vi "FlexMag - 23-03-2023.vi"() -> ()   [LabVIEW 2018] (continued)
        n2608 = Mantissa & Exponent(0:w3782) -> (2:w3784:dbl)  [unwired: 1 out]
        n2609 = Mantissa & Exponent(0:w3768) -> (2:w3770:dbl)  [unwired: 1 out]
        n2610 = Mantissa & Exponent(0:w3822) -> (2:w3824:dbl)  [unwired: 1 out]
        n2611 = Mantissa & Exponent(0:w3819) -> (2:w3817:dbl)  [unwired: 1 out]
        n2612 = Mantissa & Exponent(0:w3867) -> (2:w3863:dbl)  [unwired: 1 out]
        n2613 = Mantissa & Exponent(0:w3833) -> (2:w3831:dbl)  [unwired: 1 out]
        n2614 = Mantissa & Exponent(0:w3837) -> (2:w3839:dbl)  [unwired: 1 out]
        n2615 = case shown="2" w3741 {
          tunnel: w3738 -> [_ w3876 _]
          tunnel: w3742 -> [_ _ w3877]
          tunnel: [u32[][] [] ("24-bit pixmap") w3876 w3877] -> w3740
          frame 0, Default {
          }
          frame 1 {
          }
          frame 2 {
          }
        }
        n2616 = case shown="1" w3723 {
          tunnel: w3722 -> [_ w3879 _]
          tunnel: w3721 -> [_ _ w3880]
          tunnel: [u32[][] [] ("24-bit pixmap") w3879 w3880] -> w3726
          frame 0, Default {
          }
          frame 1 {
          }
          frame 2 {
          }
        }
        n2617 = case shown="1" w3729 {
          tunnel: w3728 -> [_ w3882 _]
          tunnel: w3727 -> [_ _ w3883]
          tunnel: [u32[][] [] ("24-bit pixmap") w3882 w3883] -> w3732
          frame 0, Default {
          }
          frame 1 {
          }
          frame 2 {
          }
        }
        n2618 = case shown="1" w3687 {
          tunnel: w3686 -> [_ w3885 _]
          tunnel: w3685 -> [_ _ w3886]
          tunnel: [u32[][] [] ("24-bit pixmap") w3885 w3886] -> w3690
          frame 0, Default {
          }
          frame 1 {
          }
          frame 2 {
          }
        }
        n2619 = case shown="1" w3694 {
          tunnel: w3695 -> [_ w3888 _]
          tunnel: w3696 -> [_ _ w3889]
          tunnel: [u32[][] [] ("24-bit pixmap") w3888 w3889] -> w3691
          frame 0, Default {
          }
          frame 1 {
          }
          frame 2 {
          }
        }
        n2620 = case shown="1" w3680 {
          tunnel: w3681 -> [_ w3891 _]
          tunnel: w3682 -> [_ _ w3892]
          tunnel: [u32[][] [] ("24-bit pixmap") w3891 w3892] -> w3677
          frame 0, Default {
          }
          frame 1 {
          }
          frame 2 {
          }
        }
        n2621 = case shown="1" w3857 {
          tunnel: w3858 -> [_ w3924 _]
          tunnel: w3859 -> [_ _ w3925]
          tunnel: [u32[][] [] ("24-bit pixmap") w3924 w3925] -> w3852
          frame 0, Default {
          }
          frame 1 {
          }
          frame 2 {
          }
        }
        n2622 = case shown="1" w3673 {
          tunnel: w3672 -> [_ w3894 _]
          tunnel: w3671 -> [_ _ w3895]
          tunnel: [u32[][] [] ("24-bit pixmap") w3894 w3895] -> w3676
          frame 0, Default {
          }
          frame 1 {
          }
          frame 2 {
          }
        }
        n2623 = case shown="2" w3744 {
          tunnel: w3749 -> [_ w3897 _]
          tunnel: w3743 -> [_ _ w3898]
          tunnel: [u32[][] [] ("24-bit pixmap") w3897 w3898] -> w3747
          frame 0, Default {
          }
          frame 1 {
          }
          frame 2 {
          }
        }
        n2624 = case shown="1" w3777 {
          tunnel: w3776 -> [_ w3903 _]
          tunnel: w3775 -> [_ _ w3904]
          tunnel: [u32[][] [] ("24-bit pixmap") w3903 w3904] -> w3780
          frame 0, Default {
          }
          frame 1 {
          }
          frame 2 {
          }
        }
        n2625 = case shown="1" w3762 {
          tunnel: w3763 -> [_ w3900 _]
          tunnel: w3764 -> [_ _ w3901]
          tunnel: [u32[][] [] ("24-bit pixmap") w3900 w3901] -> w3759
          frame 0, Default {
          }
          frame 1 {
          }
          frame 2 {
          }
        }
        n2626 = case shown="1" w3784 {
          tunnel: w3785 -> [_ w3906 _]
          tunnel: w3786 -> [_ _ w3907]
          tunnel: [u32[][] [] ("24-bit pixmap") w3906 w3907] -> w3781
          frame 0, Default {
          }
          frame 1 {
          }
          frame 2 {
          }
        }
        n2627 = case shown="1" w3770 {
          tunnel: w3771 -> [_ w3909 _]
          tunnel: w3772 -> [_ _ w3910]
          tunnel: [u32[][] [] ("24-bit pixmap") w3909 w3910] -> w3767
          frame 0, Default {
          }
          frame 1 {
          }
          frame 2 {
          }
        }
        n2628 = case shown="1" w3824 {
          tunnel: w3825 -> [_ w3912 _]
          tunnel: w3826 -> [_ _ w3913]
          tunnel: [u32[][] [] ("24-bit pixmap") w3912 w3913] -> w3821
          frame 0, Default {
          }
          frame 1 {
          }
          frame 2 {
          }
        }
        n2629 = case shown="1" w3817 {
          tunnel: w3816 -> [_ w3915 _]
          tunnel: w3815 -> [_ _ w3916]
          tunnel: [u32[][] [] ("24-bit pixmap") w3915 w3916] -> w3820
          frame 0, Default {
          }
          frame 1 {
          }
          frame 2 {
          }
        }
        n2630 = case shown="1" w3863 {
          tunnel: w3862 -> [_ w3927 _]
          tunnel: w3861 -> [_ _ w3928]
          tunnel: [u32[][] [] ("24-bit pixmap") w3927 w3928] -> w3868
          frame 0, Default {
          }
          frame 1 {
          }
          frame 2 {
          }
        }
        n2631 = case shown="1" w3831 {
          tunnel: w3830 -> [_ w3918 _]
          tunnel: w3829 -> [_ _ w3919]
          tunnel: [u32[][] [] ("24-bit pixmap") w3918 w3919] -> w3834
          frame 0, Default {
          }
          frame 1 {
          }
          frame 2 {
          }
        }
        n2632 = case shown="1" w3839 {
          tunnel: w3840 -> [_ w3921 _]
          tunnel: w3841 -> [_ _ w3922]
          tunnel: [u32[][] [] ("24-bit pixmap") w3921 w3922] -> w3836
          frame 0, Default {
          }
          frame 1 {
          }
          frame 2 {
          }
        }
        n2633 = call-poly <vilib>:"Draw Unflattened Pixmap.vi"("top left point(0, 0)"=cluster{"x":i16, "y":i16} {"x"=80, "y"=180}, "data (RGB format)"=w3871) -> ("new picture"=w3851:picture)  [unwired: 7 in]
        n2634 = call-poly <vilib>:"Draw Unflattened Pixmap.vi"("top left point(0, 0)"=cluster{"x":i16, "y":i16} {"x"=80, "y"=180}, "data (RGB format)"=w3872) -> ("new picture"=→"CH4 front main":picture)  [unwired: 7 in]
        n2635 = call-poly <vilib>:"Draw Unflattened Pixmap.vi"("top left point(0, 0)"=cluster{"x":i16, "y":i16} {"x"=80, "y"=180}, "data (RGB format)"=w3874) -> ("new picture"=→"CH3 front main":picture)  [unwired: 7 in]
        n2636 = call-poly <vilib>:"Draw Unflattened Pixmap.vi"("top left point(0, 0)"=cluster{"x":i16, "y":i16} {"x"=80, "y"=180}, "data (RGB format)"=w3873) -> ("new picture"=w3860:picture)  [unwired: 7 in]
        n2637 = call-poly <vilib>:"Draw Unflattened Pixmap.vi"("picture"=w3860, "top left point(0, 0)"=cluster{"x":i16, "y":i16} {"x"=492, "y"=218}, "data (RGB format)"=w3868) -> ("new picture"=w3835:picture)  [unwired: 6 in]
        n2638 = call-poly <vilib>:"Draw Unflattened Pixmap.vi"("picture"=w3835, "top left point(0, 0)"=cluster{"x":i16, "y":i16} {"x"=258, "y"=636}, "data (RGB format)"=w3836) -> ("new picture"=w3812:picture)  [unwired: 6 in]
        n2639 = call-poly <vilib>:"Draw Unflattened Pixmap.vi"("picture"=w3812, "top left point(0, 0)"=cluster{"x":i16, "y":i16} {"x"=350, "y"=648}, "data (RGB format)"=w3834) -> ("new picture"=w3813:picture)  [unwired: 6 in]
        n2640 = call-poly <vilib>:"Draw Unflattened Pixmap.vi"("picture"=w3813, "top left point(0, 0)"=cluster{"x":i16, "y":i16} {"x"=184, "y"=632}, "data (RGB format)"=w3820) -> ("new picture"=w3811:picture)  [unwired: 6 in]
        n2641 = call-poly <vilib>:"Draw Unflattened Pixmap.vi"("picture"=w3811, "top left point(0, 0)"=cluster{"x":i16, "y":i16} {"x"=464, "y"=654}, "data (RGB format)"=w3821) -> ("new picture"=w3766:picture)  [unwired: 6 in]
        n2642 = call-poly <vilib>:"Draw Unflattened Pixmap.vi"("picture"=w3766, "top left point(0, 0)"=cluster{"x":i16, "y":i16} {"x"=360, "y"=686}, "data (RGB format)"=w3767) -> ("new picture"=w3788:picture)  [unwired: 6 in]
        n2643 = call-poly <vilib>:"Draw Unflattened Pixmap.vi"("picture"=w3788, "top left point(0, 0)"=cluster{"x":i16, "y":i16} {"x"=474, "y"=298}, "data (RGB format)"=w3781) -> ("new picture"=w3789:picture)  [unwired: 6 in]
        n2644 = call-poly <vilib>:"Draw Unflattened Pixmap.vi"("picture"=w3789, "top left point(0, 0)"=cluster{"x":i16, "y":i16} {"x"=160, "y"=298}, "data (RGB format)"=w3780) -> ("new picture"=w3755:picture)  [unwired: 6 in]
        n2645 = call-poly <vilib>:"Draw Unflattened Pixmap.vi"("picture"=w3755, "top left point(0, 0)"=cluster{"x":i16, "y":i16} {"x"=554, "y"=362}, "data (RGB format)"=w3759) -> ("new picture"=w3746:picture)  [unwired: 6 in]
        n2646 = call-poly <vilib>:"Draw Unflattened Pixmap.vi"("picture"=w3746, "top left point(0, 0)"=cluster{"x":i16, "y":i16} {"x"=80, "y"=362}, "data (RGB format)"=w3747) -> ("new picture"=→"CH3 top main":picture)  [unwired: 6 in]
        n2647 = call-poly <vilib>:"Draw Unflattened Pixmap.vi"("picture"=w3851, "top left point(0, 0)"=cluster{"x":i16, "y":i16} {"x"=440, "y"=216}, "data (RGB format)"=w3852) -> ("new picture"=w3668:picture)  [unwired: 6 in]
        n2648 = call-poly <vilib>:"Draw Unflattened Pixmap.vi"("picture"=w3668, "top left point(0, 0)"=cluster{"x":i16, "y":i16} {"x"=208, "y"=636}, "data (RGB format)"=w3676) -> ("new picture"=w3699:picture)  [unwired: 6 in]
        n2649 = call-poly <vilib>:"Draw Unflattened Pixmap.vi"("picture"=w3699, "top left point(0, 0)"=cluster{"x":i16, "y":i16} {"x"=300, "y"=644}, "data (RGB format)"=w3677) -> ("new picture"=w3698:picture)  [unwired: 6 in]
        n2650 = call-poly <vilib>:"Draw Unflattened Pixmap.vi"("picture"=w3698, "top left point(0, 0)"=cluster{"x":i16, "y":i16} {"x"=134, "y"=632}, "data (RGB format)"=w3691) -> ("new picture"=w3700:picture)  [unwired: 6 in]
        n2651 = call-poly <vilib>:"Draw Unflattened Pixmap.vi"("picture"=w3700, "top left point(0, 0)"=cluster{"x":i16, "y":i16} {"x"=414, "y"=654}, "data (RGB format)"=w3690) -> ("new picture"=w3667:picture)  [unwired: 6 in]
        n2652 = call-poly <vilib>:"Draw Unflattened Pixmap.vi"("picture"=w3667, "top left point(0, 0)"=cluster{"x":i16, "y":i16} {"x"=310, "y"=688}, "data (RGB format)"=w3732) -> ("new picture"=w3719:picture)  [unwired: 6 in]
        n2653 = call-poly <vilib>:"Draw Unflattened Pixmap.vi"("picture"=w3719, "top left point(0, 0)"=cluster{"x":i16, "y":i16} {"x"=424, "y"=298}, "data (RGB format)"=w3726) -> ("new picture"=w3665:picture)  [unwired: 6 in]
        n2654 = call-poly <vilib>:"Draw Unflattened Pixmap.vi"("picture"=w3665, "top left point(0, 0)"=cluster{"x":i16, "y":i16} {"x"=504, "y"=362}, "data (RGB format)"=w3740) -> ("new picture"=→"CH4 top main":picture)  [unwired: 6 in]
      }
      frame #4 {
        # "ch atm4"
        # "ch atm3"
        # "ch atm2"
        # "ch atm1"
        # "ch bg4"
        # "ch bg3"
        # "ch bg2"
        # "ch bg1"
        # "ch pg4"
        # "ch pg3"
        # "ch pg2"
        # "ch pg1"
        # "pl atm1"
        # "pl atm2"
        # "pl atm3"
        # "pl atm4"
        # "pl pg4"
        # "pl pg3"
        # "pl pg2"
        # "pl pg1"
        n2655 = local read "Mouse Position"() -> (w4017:cluster{"X":i32, "Y":i32})
        n2656 = local read "Mouse .Button"() -> (w4036:bool)
        n2657 = Unbundle By Name(w4017) -> ("X"=w4213:i32, "Y"=w4214:i32)
        n2658 = In Range and Coerce(upper limit=542, x=w4213, lower limit=452 ("upper limit")) -> (In Range?=w4399:bool)  [unwired: 1 out]
        n2659 = In Range and Coerce(upper limit=120, x=w4214, lower limit=28 ("upper limit")) -> (In Range?=w4400:bool)  [unwired: 1 out]
        n2660 = In Range and Coerce(upper limit=1190, x=w4213, lower limit=1100 ("upper limit")) -> (In Range?=w4390:bool)  [unwired: 1 out]
        n2661 = In Range and Coerce(upper limit=120, x=w4214, lower limit=28 ("upper limit")) -> (In Range?=w4389:bool)  [unwired: 1 out]
        n2662 = In Range and Coerce(upper limit=452, x=w4213, lower limit=424 ("upper limit")) -> (In Range?=w4367:bool)  [unwired: 1 out]
        n2663 = In Range and Coerce(upper limit=198, x=w4214, lower limit=142 ("upper limit")) -> (In Range?=w4366:bool)  [unwired: 1 out]
        n2664 = In Range and Coerce(upper limit=1110, x=w4213, lower limit=1074 ("upper limit")) -> (In Range?=w4375:bool)  [unwired: 1 out]
        n2665 = In Range and Coerce(upper limit=198, x=w4214, lower limit=142 ("upper limit")) -> (In Range?=w4376:bool)  [unwired: 1 out]
        n2666 = In Range and Coerce(upper limit=568, x=w4213, lower limit=530 ("upper limit")) -> (In Range?=w4350:bool)  [unwired: 1 out]
        n2667 = In Range and Coerce(upper limit=180, x=w4214, lower limit=146 ("upper limit")) -> (In Range?=w4351:bool)  [unwired: 1 out]
        n2668 = In Range and Coerce(upper limit=1216, x=w4213, lower limit=1182 ("upper limit")) -> (In Range?=w4342:bool)  [unwired: 1 out]
        n2669 = In Range and Coerce(upper limit=180, x=w4214, lower limit=146 ("upper limit")) -> (In Range?=w4341:bool)  [unwired: 1 out]
        n2670 = In Range and Coerce(upper limit=550, x=w4213, lower limit=510 ("upper limit")) -> (In Range?=w4319:bool)  [unwired: 1 out]
        n2671 = In Range and Coerce(upper limit=264, x=w4214, lower limit=210 ("upper limit")) -> (In Range?=w4318:bool)  [unwired: 1 out]
        n2672 = In Range and Coerce(upper limit=1200, x=w4213, lower limit=1164 ("upper limit")) -> (In Range?=w4327:bool)  [unwired: 1 out]
        n2673 = In Range and Coerce(upper limit=264, x=w4214, lower limit=210 ("upper limit")) -> (In Range?=w4328:bool)  [unwired: 1 out]
        n2674 = In Range and Coerce(upper limit=508, x=w4213, lower limit=468 ("upper limit")) -> (In Range?=w4302:bool)  [unwired: 1 out]
        n2675 = In Range and Coerce(upper limit=350, x=w4214, lower limit=320 ("upper limit")) -> (In Range?=w4303:bool)  [unwired: 1 out]
        n2676 = In Range and Coerce(upper limit=1160, x=w4213, lower limit=1118 ("upper limit")) -> (In Range?=w4294:bool)  [unwired: 1 out]
        n2677 = In Range and Coerce(upper limit=350, x=w4214, lower limit=320 ("upper limit")) -> (In Range?=w4293:bool)  [unwired: 1 out]
        n2678 = In Range and Coerce(upper limit=536, x=w4213, lower limit=452 ("upper limit")) -> (In Range?=w4271:bool)  [unwired: 1 out]
        n2679 = In Range and Coerce(upper limit=458, x=w4214, lower limit=392 ("upper limit")) -> (In Range?=w4270:bool)  [unwired: 1 out]
        n2680 = In Range and Coerce(upper limit=1188, x=w4213, lower limit=1106 ("upper limit")) -> (In Range?=w4279:bool)  [unwired: 1 out]
        n2681 = In Range and Coerce(upper limit=458, x=w4214, lower limit=392 ("upper limit")) -> (In Range?=w4280:bool)  [unwired: 1 out]
        n2682 = In Range and Coerce(upper limit=434, x=w4213, lower limit=408 ("upper limit")) -> (In Range?=w4254:bool)  [unwired: 1 out]
        n2683 = In Range and Coerce(upper limit=452, x=w4214, lower limit=398 ("upper limit")) -> (In Range?=w4255:bool)  [unwired: 1 out]
        n2684 = In Range and Coerce(upper limit=1084, x=w4213, lower limit=1058 ("upper limit")) -> (In Range?=w4246:bool)  [unwired: 1 out]
        n2685 = In Range and Coerce(upper limit=452, x=w4214, lower limit=398 ("upper limit")) -> (In Range?=w4245:bool)  [unwired: 1 out]
        n2686 = In Range and Coerce(upper limit=546, x=w4213, lower limit=456 ("upper limit")) -> (In Range?=w4223:bool)  [unwired: 1 out]
        n2687 = In Range and Coerce(upper limit=488, x=w4214, lower limit=460 ("upper limit")) -> (In Range?=w4222:bool)  [unwired: 1 out]
        n2688 = In Range and Coerce(upper limit=1196, x=w4213, lower limit=1108 ("upper limit")) -> (In Range?=w4231:bool)  [unwired: 1 out]
        n2689 = In Range and Coerce(upper limit=488, x=w4214, lower limit=460 ("upper limit")) -> (In Range?=w4232:bool)  [unwired: 1 out]
        n2690 = In Range and Coerce(upper limit=214, x=w4213, lower limit=124 ("upper limit")) -> (In Range?=w4402:bool)  [unwired: 1 out]
        n2691 = In Range and Coerce(upper limit=120, x=w4214, lower limit=28 ("upper limit")) -> (In Range?=w4401:bool)  [unwired: 1 out]
        n2692 = In Range and Coerce(upper limit=866, x=w4213, lower limit=778 ("upper limit")) -> (In Range?=w4387:bool)  [unwired: 1 out]
        n2693 = In Range and Coerce(upper limit=120, x=w4214, lower limit=28 ("upper limit")) -> (In Range?=w4388:bool)  [unwired: 1 out]
        n2694 = In Range and Coerce(upper limit=124, x=w4213, lower limit=98 ("upper limit")) -> (In Range?=w4364:bool)  [unwired: 1 out]
        n2695 = In Range and Coerce(upper limit=198, x=w4214, lower limit=142 ("upper limit")) -> (In Range?=w4365:bool)  [unwired: 1 out]
        n2696 = In Range and Coerce(upper limit=776, x=w4213, lower limit=750 ("upper limit")) -> (In Range?=w4378:bool)  [unwired: 1 out]
        n2697 = In Range and Coerce(upper limit=198, x=w4214, lower limit=142 ("upper limit")) -> (In Range?=w4377:bool)  [unwired: 1 out]
        n2698 = In Range and Coerce(upper limit=242, x=w4213, lower limit=206 ("upper limit")) -> (In Range?=w4353:bool)  [unwired: 1 out]
        n2699 = In Range and Coerce(upper limit=180, x=w4214, lower limit=146 ("upper limit")) -> (In Range?=w4352:bool)  [unwired: 1 out]
        n2700 = In Range and Coerce(upper limit=894, x=w4213, lower limit=856 ("upper limit")) -> (In Range?=w4339:bool)  [unwired: 1 out]
        n2701 = In Range and Coerce(upper limit=180, x=w4214, lower limit=146 ("upper limit")) -> (In Range?=w4340:bool)  [unwired: 1 out]
        n2702 = In Range and Coerce(upper limit=224, x=w4213, lower limit=186 ("upper limit")) -> (In Range?=w4316:bool)  [unwired: 1 out]
        n2703 = In Range and Coerce(upper limit=264, x=w4214, lower limit=210 ("upper limit")) -> (In Range?=w4317:bool)  [unwired: 1 out]
        n2704 = In Range and Coerce(upper limit=876, x=w4213, lower limit=842 ("upper limit")) -> (In Range?=w4330:bool)  [unwired: 1 out]
        n2705 = In Range and Coerce(upper limit=264, x=w4214, lower limit=210 ("upper limit")) -> (In Range?=w4329:bool)  [unwired: 1 out]
        n2706 = In Range and Coerce(upper limit=182, x=w4213, lower limit=140 ("upper limit")) -> (In Range?=w4305:bool)  [unwired: 1 out]
        n2707 = In Range and Coerce(upper limit=350, x=w4214, lower limit=320 ("upper limit")) -> (In Range?=w4304:bool)  [unwired: 1 out]
        n2708 = In Range and Coerce(upper limit=836, x=w4213, lower limit=794 ("upper limit")) -> (In Range?=w4291:bool)  [unwired: 1 out]
        n2709 = In Range and Coerce(upper limit=350, x=w4214, lower limit=320 ("upper limit")) -> (In Range?=w4292:bool)  [unwired: 1 out]
        n2710 = In Range and Coerce(upper limit=210, x=w4213, lower limit=126 ("upper limit")) -> (In Range?=w4268:bool)  [unwired: 1 out]
        n2711 = In Range and Coerce(upper limit=458, x=w4214, lower limit=392 ("upper limit")) -> (In Range?=w4269:bool)  [unwired: 1 out]
        n2712 = In Range and Coerce(upper limit=862, x=w4213, lower limit=778 ("upper limit")) -> (In Range?=w4282:bool)  [unwired: 1 out]
        n2713 = In Range and Coerce(upper limit=458, x=w4214, lower limit=392 ("upper limit")) -> (In Range?=w4281:bool)  [unwired: 1 out]
        n2714 = In Range and Coerce(upper limit=108, x=w4213, lower limit=82 ("upper limit")) -> (In Range?=w4257:bool)  [unwired: 1 out]
        n2715 = In Range and Coerce(upper limit=452, x=w4214, lower limit=398 ("upper limit")) -> (In Range?=w4256:bool)  [unwired: 1 out]
        n2716 = In Range and Coerce(upper limit=758, x=w4213, lower limit=734 ("upper limit")) -> (In Range?=w4243:bool)  [unwired: 1 out]
        n2717 = In Range and Coerce(upper limit=452, x=w4214, lower limit=398 ("upper limit")) -> (In Range?=w4244:bool)  [unwired: 1 out]
        n2718 = In Range and Coerce(upper limit=218, x=w4213, lower limit=130 ("upper limit")) -> (In Range?=w4220:bool)  [unwired: 1 out]
        n2719 = In Range and Coerce(upper limit=488, x=w4214, lower limit=460 ("upper limit")) -> (In Range?=w4221:bool)  [unwired: 1 out]
        n2720 = In Range and Coerce(upper limit=872, x=w4213, lower limit=782 ("upper limit")) -> (In Range?=w4234:bool)  [unwired: 1 out]
        n2721 = In Range and Coerce(upper limit=488, x=w4214, lower limit=460 ("upper limit")) -> (In Range?=w4233:bool)  [unwired: 1 out]
        n2722 = And(x=w4399, y=w4400) -> (x .and. y?=w4034:bool)
        n2723 = And(x=w4390, y=w4389) -> (x .and. y?=w4032:bool)
        n2724 = And(x=w4367, y=w4366) -> (x .and. y?=w4030:bool)
        n2725 = And(x=w4375, y=w4376) -> (x .and. y?=w4028:bool)
        n2726 = And(x=w4350, y=w4351) -> (x .and. y?=w4026:bool)
        n2727 = And(x=w4342, y=w4341) -> (x .and. y?=w4023:bool)
        n2728 = And(x=w4319, y=w4318) -> (x .and. y?=w4021:bool)
        n2729 = And(x=w4327, y=w4328) -> (x .and. y?=w4019:bool)
        n2730 = And(x=w4302, y=w4303) -> (x .and. y?=w4016:bool)
        n2731 = And(x=w4294, y=w4293) -> (x .and. y?=w4014:bool)
        n2732 = And(x=w4271, y=w4270) -> (x .and. y?=w4012:bool)
        n2733 = And(x=w4279, y=w4280) -> (x .and. y?=w4010:bool)
        n2734 = And(x=w4254, y=w4255) -> (x .and. y?=w4008:bool)
        n2735 = And(x=w4246, y=w4245) -> (x .and. y?=w4006:bool)
        n2736 = And(x=w4223, y=w4222) -> (x .and. y?=w4004:bool)
        n2737 = And(x=w4231, y=w4232) -> (x .and. y?=w4000:bool)
        n2738 = And(x=w4402, y=w4401) -> (x .and. y?=w4035:bool)
        n2739 = And(x=w4387, y=w4388) -> (x .and. y?=w4033:bool)
        n2740 = And(x=w4364, y=w4365) -> (x .and. y?=w4031:bool)
        n2741 = And(x=w4378, y=w4377) -> (x .and. y?=w4029:bool)
        n2742 = And(x=w4353, y=w4352) -> (x .and. y?=w4027:bool)
        n2743 = And(x=w4339, y=w4340) -> (x .and. y?=w4024:bool)
        n2744 = And(x=w4316, y=w4317) -> (x .and. y?=w4022:bool)
        n2745 = And(x=w4330, y=w4329) -> (x .and. y?=w4020:bool)
        n2746 = And(x=w4305, y=w4304) -> (x .and. y?=w4018:bool)
        n2747 = And(x=w4291, y=w4292) -> (x .and. y?=w4015:bool)
        n2748 = And(x=w4268, y=w4269) -> (x .and. y?=w4013:bool)
        n2749 = And(x=w4282, y=w4281) -> (x .and. y?=w4011:bool)
        n2750 = And(x=w4257, y=w4256) -> (x .and. y?=w4009:bool)
        n2751 = And(x=w4243, y=w4244) -> (x .and. y?=w4007:bool)
        n2752 = And(x=w4220, y=w4221) -> (x .and. y?=w4005:bool)
        n2753 = And(x=w4234, y=w4233) -> (x .and. y?=w4003:bool)
        n2754 = And(x=w4036, y=w4034) -> (x .and. y?=w3968:bool)
        n2755 = And(x=w4036, y=w4032) -> (x .and. y?=w3966:bool)
        n2756 = And(x=w4036, y=w4030) -> (x .and. y?=w3964:bool)
        n2757 = And(x=w4036, y=w4028) -> (x .and. y?=w3962:bool)
        n2758 = And(x=w4036, y=w4016) -> (x .and. y?=w3960:bool)
        n2759 = And(x=w4036, y=w4014) -> (x .and. y?=w3958:bool)
        n2760 = And(x=w4036, y=w4012) -> (x .and. y?=w3956:bool)
        n2761 = And(x=w4036, y=w4010) -> (x .and. y?=w3954:bool)
        n2762 = And(x=w4036, y=w4008) -> (x .and. y?=w3952:bool)
        n2763 = And(x=w4036, y=w4006) -> (x .and. y?=w3950:bool)
        n2764 = And(x=w4036, y=w4004) -> (x .and. y?=w3948:bool)
        n2765 = And(x=w4036, y=w4000) -> (x .and. y?=w3946:bool)
        n2766 = And(x=w4036, y=w4035) -> (x .and. y?=w3969:bool)
        n2767 = And(x=w4036, y=w4033) -> (x .and. y?=w3967:bool)
        n2768 = And(x=w4036, y=w4031) -> (x .and. y?=w3965:bool)
        n2769 = And(x=w4036, y=w4029) -> (x .and. y?=w3963:bool)
        n2770 = And(x=w4036, y=w4018) -> (x .and. y?=w3961:bool)
        n2771 = And(x=w4036, y=w4015) -> (x .and. y?=w3959:bool)
        n2772 = And(x=w4036, y=w4013) -> (x .and. y?=w3957:bool)
        n2773 = And(x=w4036, y=w4011) -> (x .and. y?=w3955:bool)
        n2774 = And(x=w4036, y=w4009) -> (x .and. y?=w3953:bool)
        n2775 = And(x=w4036, y=w4007) -> (x .and. y?=w3951:bool)
        n2776 = And(x=w4036, y=w4005) -> (x .and. y?=w3949:bool)
        n2777 = And(x=w4036, y=w4003) -> (x .and. y?=w3947:bool)
        n2778 = case shown="True" w3966 {
          frame False {
          }
          frame True {
            "ch1 mp timer" <- TRUE ("ch1 mp timer")
          }
        }
        n2779 = case shown="True" w3950 {
          frame False {
          }
          frame True {
            "ch1 ch vbv timer" <- TRUE ("ch1 tp vbv timer")
          }
        }
        n2780 = case shown="True" w3968 {
          frame False {
          }
          frame True {
            "ch3 mp timer" <- TRUE ("ch3 mp timer")
          }
        }
        n2781 = case shown="True" w3964 {
          frame False {
          }
          frame True {
            "ch3 pl vbv timer" <- TRUE ("ch3 pl vbv timer")
          }
        }
        n2782 = case shown="True" w3969 {
          frame False {
          }
          frame True {
            "ch4 mp timer" <- TRUE ("ch4 mp timer")
          }
        }
        n2783 = case shown="True" w3967 {
          frame False {
          }
          frame True {
            "ch2 mp timer" <- TRUE ("ch2 mp timer")
          }
        }
        n2784 = case shown="True" w3965 {
          frame False {
          }
          frame True {
            "ch4 pl vbv timer" <- TRUE ("ch4 pl vbv timer")
          }
        }
        n2785 = case shown="True" w3961 {
          frame False {
          }
          frame True {
            "ch4 tp bv timer" <- TRUE ("ch4 tp bv timer")
          }
        }
        n2786 = case shown="True" w3946 {
          frame False {
          }
          frame True {
            "ch1 pc gv timer" <- TRUE ("ch1 pc gv timer")
          }
        }
        n2787 = case shown="True" w3963 {
          frame False {
          }
          frame True {
            "ch2 pl vbv timer" <- TRUE ("ch2 pl vbv timer")
          }
        }
        n2788 = case shown="True" w3962 {
          frame False {
          }
          frame True {
            "ch1 pl vbv timer" <- TRUE ("ch1 pl vbv timer")
          }
        }
        n2789 = case shown="True" w3960 {
          frame False {
          }
          frame True {
            "ch3 tp bv timer" <- TRUE ("ch3 tp bv timer")
          }
        }
        n2790 = case shown="True" w3949 {
          frame False {
          }
          frame True {
            "ch4 pc gv timer" <- TRUE ("ch4 pc gv timer")
          }
        }
        n2791 = case shown="True" w3952 {
          frame False {
          }
          frame True {
            "ch3 ch vbv timer" <- TRUE ("ch3 tp vbv timer")
          }
        }
        n2792 = case shown="True" w3951 {
          frame False {
          }
          frame True {
            "ch2 ch vbv timer" <- TRUE ("ch2 tp vbv timer")
          }
        }
        n2793 = case shown="True" w3947 {
          frame False {
          }
          frame True {
            "ch2 pc gv timer" <- TRUE ("ch2 pc gv timer")
          }
        }
        n2794 = case shown="True" w3959 {
          frame False {
          }
          frame True {
            "ch2 tp bv timer" <- TRUE ("ch2 tp bv timer")
          }
        }
        n2795 = case shown="True" w3958 {
          frame False {
          }
          frame True {
            "ch1 tp bv timer" <- TRUE ("ch1 tp bv timer")
          }
        }
        n2796 = case shown="True" w3948 {
          frame False {
          }
          frame True {
            "ch3 pc gv timer" <- TRUE ("ch3 pc gv timer")
          }
        }
        n2797 = case shown="True" w3953 {
          frame False {
          }
          frame True {
            "ch4 ch vbv timer" <- TRUE ("ch4 tp vbv timer")
          }
        }
        n2798 = case shown="True" w3957 {
          frame False {
          }
          frame True {
            "ch4 tp timer" <- TRUE ("ch4 tp timer")
          }
        }
        n2799 = case shown="True" w3956 {
          frame False {
          }
          frame True {
            "ch3 tp timer" <- TRUE ("ch3 tp timer")
          }
        }
        n2800 = case shown="True" w3954 {
          frame False {
          }
          frame True {
            "ch1 tp timer" <- TRUE ("ch1 tp timer")
          }
        }
        n2801 = case shown="True" w3955 {
          frame False {
          }
          frame True {
            "ch2 tp timer" <- TRUE ("ch2 tp timer")
          }
        }
        n2802 = Unbundle By Name(w4017) -> ("X"=w4037:i32, "Y"=w4038:i32)
        n2803 = In Range and Coerce(upper limit=682, x=w4037, lower limit=632 ("upper limit")) -> (In Range?=w4085:bool)  [unwired: 1 out]
        n2804 = In Range and Coerce(upper limit=670, x=w4038, lower limit=534 ("upper limit")) -> (In Range?=w4086:bool)  [unwired: 1 out]
        n2805 = In Range and Coerce(upper limit=922, x=w4037, lower limit=888 ("upper limit")) -> (In Range?=w4064:bool)  [unwired: 1 out]
        n2806 = In Range and Coerce(upper limit=500, x=w4038, lower limit=464 ("upper limit")) -> (In Range?=w4063:bool)  [unwired: 1 out]
        n2807 = In Range and Coerce(upper limit=428, x=w4037, lower limit=394 ("upper limit")) -> (In Range?=w4049:bool)  [unwired: 1 out]
        n2808 = In Range and Coerce(upper limit=500, x=w4038, lower limit=464 ("upper limit")) -> (In Range?=w4050:bool)  [unwired: 1 out]
        n2809 = In Range and Coerce(upper limit=540, x=w4037, lower limit=510 ("upper limit")) -> (In Range?=w4133:bool)  [unwired: 1 out]
        n2810 = In Range and Coerce(upper limit=790, x=w4038, lower limit=760 ("upper limit")) -> (In Range?=w4134:bool)  [unwired: 1 out]
        n2811 = In Range and Coerce(upper limit=1192, x=w4037, lower limit=1162 ("upper limit")) -> (In Range?=w4124:bool)  [unwired: 1 out]
        n2812 = In Range and Coerce(upper limit=790, x=w4038, lower limit=760 ("upper limit")) -> (In Range?=w4123:bool)  [unwired: 1 out]
        n2813 = In Range and Coerce(upper limit=634, x=w4037, lower limit=584 ("upper limit")) -> (In Range?=w4100:bool)  [unwired: 1 out]
        n2814 = In Range and Coerce(upper limit=758, x=w4038, lower limit=696 ("upper limit")) -> (In Range?=w4099:bool)  [unwired: 1 out]
        n2815 = In Range and Coerce(upper limit=1286, x=w4037, lower limit=1236 ("upper limit")) -> (In Range?=w4109:bool)  [unwired: 1 out]
        n2816 = In Range and Coerce(upper limit=758, x=w4038, lower limit=696 ("upper limit")) -> (In Range?=w4110:bool)  [unwired: 1 out]
        n2817 = In Range and Coerce(upper limit=414, x=w4037, lower limit=384 ("upper limit")) -> (In Range?=w4196:bool)  [unwired: 1 out]
        n2818 = In Range and Coerce(upper limit=736, x=w4038, lower limit=708 ("upper limit")) -> (In Range?=w4195:bool)  [unwired: 1 out]
        n2819 = In Range and Coerce(upper limit=1064, x=w4037, lower limit=1036 ("upper limit")) -> (In Range?=w4205:bool)  [unwired: 1 out]
        n2820 = In Range and Coerce(upper limit=736, x=w4038, lower limit=708 ("upper limit")) -> (In Range?=w4206:bool)  [unwired: 1 out]
        n2821 = In Range and Coerce(upper limit=476, x=w4037, lower limit=438 ("upper limit")) -> (In Range?=w4181:bool)  [unwired: 1 out]
        n2822 = In Range and Coerce(upper limit=754, x=w4038, lower limit=706 ("upper limit")) -> (In Range?=w4182:bool)  [unwired: 1 out]
        n2823 = In Range and Coerce(upper limit=1128, x=w4037, lower limit=1090 ("upper limit")) -> (In Range?=w4172:bool)  [unwired: 1 out]
        n2824 = In Range and Coerce(upper limit=754, x=w4038, lower limit=706 ("upper limit")) -> (In Range?=w4171:bool)  [unwired: 1 out]
        n2825 = In Range and Coerce(upper limit=540, x=w4037, lower limit=500 ("upper limit")) -> (In Range?=w4148:bool)  [unwired: 1 out]
        n2826 = In Range and Coerce(upper limit=744, x=w4038, lower limit=710 ("upper limit")) -> (In Range?=w4147:bool)  [unwired: 1 out]
        n2827 = In Range and Coerce(upper limit=1192, x=w4037, lower limit=1152 ("upper limit")) -> (In Range?=w4157:bool)  [unwired: 1 out]
        n2828 = In Range and Coerce(upper limit=744, x=w4038, lower limit=710 ("upper limit")) -> (In Range?=w4158:bool)  [unwired: 1 out]
        n2829 = In Range and Coerce(upper limit=356, x=w4037, lower limit=306 ("upper limit")) -> (In Range?=w4088:bool)  [unwired: 1 out]
        n2830 = In Range and Coerce(upper limit=670, x=w4038, lower limit=534 ("upper limit")) -> (In Range?=w4087:bool)  [unwired: 1 out]
        n2831 = In Range and Coerce(upper limit=1010, x=w4037, lower limit=960 ("upper limit")) -> (In Range?=w4079:bool)  [unwired: 1 out]
        n2832 = In Range and Coerce(upper limit=670, x=w4038, lower limit=534 ("upper limit")) -> (In Range?=w4080:bool)  [unwired: 1 out]
        n2833 = In Range and Coerce(upper limit=1076, x=w4037, lower limit=1044 ("upper limit")) -> (In Range?=w4061:bool)  [unwired: 1 out]
        n2834 = In Range and Coerce(upper limit=500, x=w4038, lower limit=464 ("upper limit")) -> (In Range?=w4062:bool)  [unwired: 1 out]
        n2835 = In Range and Coerce(upper limit=752, x=w4037, lower limit=720 ("upper limit")) -> (In Range?=w4070:bool)  [unwired: 1 out]
        n2836 = In Range and Coerce(upper limit=500, x=w4038, lower limit=464 ("upper limit")) -> (In Range?=w4069:bool)  [unwired: 1 out]
        n2837 = In Range and Coerce(upper limit=596, x=w4037, lower limit=552 ("upper limit")) -> (In Range?=w4052:bool)  [unwired: 1 out]
        n2838 = In Range and Coerce(upper limit=500, x=w4038, lower limit=464 ("upper limit")) -> (In Range?=w4051:bool)  [unwired: 1 out]
        n2839 = In Range and Coerce(upper limit=272, x=w4037, lower limit=236 ("upper limit")) -> (In Range?=w4043:bool)  [unwired: 1 out]
        n2840 = In Range and Coerce(upper limit=500, x=w4038, lower limit=464 ("upper limit")) -> (In Range?=w4044:bool)  [unwired: 1 out]
        n2841 = In Range and Coerce(upper limit=214, x=w4037, lower limit=184 ("upper limit")) -> (In Range?=w4136:bool)  [unwired: 1 out]
        n2842 = In Range and Coerce(upper limit=790, x=w4038, lower limit=760 ("upper limit")) -> (In Range?=w4135:bool)  [unwired: 1 out]
        n2843 = In Range and Coerce(upper limit=868, x=w4037, lower limit=838 ("upper limit")) -> (In Range?=w4121:bool)  [unwired: 1 out]
        n2844 = In Range and Coerce(upper limit=790, x=w4038, lower limit=760 ("upper limit")) -> (In Range?=w4122:bool)  [unwired: 1 out]
        n2845 = In Range and Coerce(upper limit=310, x=w4037, lower limit=260 ("upper limit")) -> (In Range?=w4097:bool)  [unwired: 1 out]
        n2846 = In Range and Coerce(upper limit=758, x=w4038, lower limit=696 ("upper limit")) -> (In Range?=w4098:bool)  [unwired: 1 out]
        n2847 = In Range and Coerce(upper limit=960, x=w4037, lower limit=910 ("upper limit")) -> (In Range?=w4112:bool)  [unwired: 1 out]
        n2848 = In Range and Coerce(upper limit=758, x=w4038, lower limit=696 ("upper limit")) -> (In Range?=w4111:bool)  [unwired: 1 out]
        n2849 = In Range and Coerce(upper limit=88, x=w4037, lower limit=60 ("upper limit")) -> (In Range?=w4193:bool)  [unwired: 1 out]
        n2850 = In Range and Coerce(upper limit=736, x=w4038, lower limit=708 ("upper limit")) -> (In Range?=w4194:bool)  [unwired: 1 out]
        n2851 = In Range and Coerce(upper limit=740, x=w4037, lower limit=710 ("upper limit")) -> (In Range?=w4208:bool)  [unwired: 1 out]
        n2852 = In Range and Coerce(upper limit=736, x=w4038, lower limit=708 ("upper limit")) -> (In Range?=w4207:bool)  [unwired: 1 out]
        n2853 = In Range and Coerce(upper limit=152, x=w4037, lower limit=112 ("upper limit")) -> (In Range?=w4184:bool)  [unwired: 1 out]
        n2854 = In Range and Coerce(upper limit=754, x=w4038, lower limit=706 ("upper limit")) -> (In Range?=w4183:bool)  [unwired: 1 out]
        n2855 = In Range and Coerce(upper limit=802, x=w4037, lower limit=764 ("upper limit")) -> (In Range?=w4169:bool)  [unwired: 1 out]
        n2856 = In Range and Coerce(upper limit=754, x=w4038, lower limit=706 ("upper limit")) -> (In Range?=w4170:bool)  [unwired: 1 out]
        n2857 = In Range and Coerce(upper limit=214, x=w4037, lower limit=174 ("upper limit")) -> (In Range?=w4145:bool)  [unwired: 1 out]
        n2858 = In Range and Coerce(upper limit=744, x=w4038, lower limit=710 ("upper limit")) -> (In Range?=w4146:bool)  [unwired: 1 out]
        n2859 = In Range and Coerce(upper limit=866, x=w4037, lower limit=826 ("upper limit")) -> (In Range?=w4160:bool)  [unwired: 1 out]
        n2860 = In Range and Coerce(upper limit=744, x=w4038, lower limit=710 ("upper limit")) -> (In Range?=w4159:bool)  [unwired: 1 out]
        n2861 = And(x=w4085, y=w4086) -> (x .and. y?=w3978:bool)
        n2862 = And(x=w4064, y=w4063) -> (x .and. y?=w3975:bool)
        n2863 = And(x=w4049, y=w4050) -> (x .and. y?=w3972:bool)
        n2864 = And(x=w4133, y=w4134) -> (x .and. y?=w3986:bool)
        n2865 = And(x=w4124, y=w4123) -> (x .and. y?=w3984:bool)
        n2866 = And(x=w4100, y=w4099) -> (x .and. y?=w3982:bool)
        n2867 = And(x=w4109, y=w4110) -> (x .and. y?=w3980:bool)
        n2868 = And(x=w4196, y=w4195) -> (x .and. y?=w3998:bool)
        n2869 = And(x=w4205, y=w4206) -> (x .and. y?=w3996:bool)
        n2870 = And(x=w4181, y=w4182) -> (x .and. y?=w3994:bool)
        n2871 = And(x=w4172, y=w4171) -> (x .and. y?=w3992:bool)
        n2872 = And(x=w4148, y=w4147) -> (x .and. y?=w3990:bool)
        n2873 = And(x=w4157, y=w4158) -> (x .and. y?=w3988:bool)
        n2874 = And(x=w4088, y=w4087) -> (x .and. y?=w3979:bool)
        n2875 = And(x=w4079, y=w4080) -> (x .and. y?=w3977:bool)
        n2876 = And(x=w4061, y=w4062) -> (x .and. y?=w3976:bool)
        n2877 = And(x=w4070, y=w4069) -> (x .and. y?=w3974:bool)
        n2878 = And(x=w4052, y=w4051) -> (x .and. y?=w3973:bool)
        n2879 = And(x=w4043, y=w4044) -> (x .and. y?=w3971:bool)
        n2880 = And(x=w4136, y=w4135) -> (x .and. y?=w3987:bool)
        n2881 = And(x=w4121, y=w4122) -> (x .and. y?=w3985:bool)
        n2882 = And(x=w4097, y=w4098) -> (x .and. y?=w3983:bool)
        n2883 = And(x=w4112, y=w4111) -> (x .and. y?=w3981:bool)
        n2884 = And(x=w4193, y=w4194) -> (x .and. y?=w3999:bool)
        n2885 = And(x=w4208, y=w4207) -> (x .and. y?=w3997:bool)
        n2886 = And(x=w4184, y=w4183) -> (x .and. y?=w3995:bool)
        n2887 = And(x=w4169, y=w4170) -> (x .and. y?=w3993:bool)
        n2888 = And(x=w4145, y=w4146) -> (x .and. y?=w3991:bool)
        n2889 = And(x=w4160, y=w4159) -> (x .and. y?=w3989:bool)
        n2890 = And(x=w4036, y=w3988) -> (x .and. y?=w3935:bool)
        n2891 = And(x=w4036, y=w3989) -> (x .and. y?=w3936:bool)
        n2892 = And(x=w4036, y=w3978) -> (x .and. y?=w3938:bool)
        n2893 = And(x=w4036, y=w3975) -> (x .and. y?=w3941:bool)
        n2894 = And(x=w4036, y=w3972) -> (x .and. y?=w3944:bool)
        n2895 = And(x=w4036, y=w3979) -> (x .and. y?=w3937:bool)
        n2896 = And(x=w4036, y=w3977) -> (x .and. y?=w3939:bool)
        n2897 = And(x=w4036, y=w3976) -> (x .and. y?=w3940:bool)
        n2898 = And(x=w4036, y=w3974) -> (x .and. y?=w3942:bool)
        n2899 = And(x=w4036, y=w3973) -> (x .and. y?=w3943:bool)
        n2900 = And(x=w4036, y=w3971) -> (x .and. y?=w3945:bool)
        n2901 = And(x=w4036, y=w3994) -> (x .and. y?=w3933:bool)
        n2902 = And(x=w4036, y=w3992) -> (x .and. y?=w3929:bool)
        n2903 = And(x=w4036, y=w3990) -> (x .and. y?=w3931:bool)
        n2904 = And(x=w4036, y=w3993) -> (x .and. y?=w3932:bool)
        n2905 = And(x=w4036, y=w3991) -> (x .and. y?=w3930:bool)
        n2906 = And(x=w4036, y=w3995) -> (x .and. y?=w3934:bool)
        n2907 = case shown="True" w3935 {
          frame False {
          }
          frame True {
            "ch1 bg bv timer" <- TRUE ("ch1 bg bv timer")
          }
        }
        n2908 = case shown="True" w3937 {
          frame False {
          }
          frame True {
            "ch3-4 trns gv timer" <- TRUE ("ch3-4 trns gv timer")
          }
        }
        n2909 = case shown="True" w3941 {
          frame False {
          }
          frame True {
            "ch2 trnsbp right timer" <- TRUE ("ch2 gv bp right timer")
          }
        }
        n2910 = case shown="True" w3944 {
          frame False {
          }
          frame True {
            "ch3 trnsbp left timer" <- TRUE ("ch3 gv bp left timer")
          }
        }
        n2911 = case shown="True" w3945 {
          frame False {
          }
          frame True {
            "ch4 trnsbp right timer" <- TRUE ("ch4 gv bp right timer")
          }
        }
        n2912 = case shown="True" w3938 {
          frame False {
          }
          frame True {
            "ch2-3 trns gv timer" <- TRUE ("ch2-3 trns gv timer")
          }
        }
        n2913 = case shown="True" w3931 {
          frame False {
          }
          frame True {
            "ch3 bg bv timer" <- TRUE ("ch3 bg bv timer")
          }
        }
        n2914 = case shown="True" w3939 {
          frame False {
          }
          frame True {
            "ch1-2 trns gv timer" <- TRUE ("ch1-2 trns gv timer")
          }
        }
        n2915 = case shown="True" w3943 {
          frame False {
          }
          frame True {
            "ch3 trnsbp right timer" <- TRUE ("ch3 gv bp right timer")
          }
        }
        n2916 = case shown="True" w3936 {
          frame False {
          }
          frame True {
            "ch2 bg bv timer" <- TRUE ("ch2 bg bv timer")
          }
        }
        n2917 = case shown="True" w3930 {
          frame False {
          }
          frame True {
            "ch4 bg bv timer" <- TRUE ("ch4 bg bv timer")
          }
        }
        n2918 = case shown="True" w3940 {
          frame False {
          }
          frame True {
            "ch1 trnsbp left timer" <- TRUE ("ch1 gv bp left timer")
          }
        }
        n2919 = case shown="True" w3933 {
          frame False {
          }
          frame True {
            "ch3 cc timer" <- TRUE ("ch3 cc timer")
          }
        }
        n2920 = case shown="True" w3929 {
          frame False {
          }
          frame True {
            "ch1 cc timer" <- TRUE ("ch1 cc timer")
          }
        }
        n2921 = case shown="True" w3942 {
          frame False {
          }
          frame True {
            "ch2 trnsbp left timer" <- TRUE ("ch2 gv bp left timer")
          }
        }
        n2922 = case shown="True" w3934 {
          frame False {
          }
          frame True {
            "ch4 cc timer" <- TRUE ("ch4 cc timer")
          }
        }
        n2923 = case shown="True" w3932 {
          frame False {
          }
          frame True {
            "ch2 cc timer" <- TRUE ("ch2 cc timer")
          }
        }
        n2924 = Build Array(FALSE, w4035, w4034, w4033, w4032, w4031, w4030, w4029, w4028, w4027, w4026, w4024, w4023, w4022, w4021, w4020, w4019, w4018, w4016, w4015, w4014, w4013, w4012, w4011, w4010, w4009, w4008, w4007, w4006, w4005, w4004, w4003) -> (w4002:bool[])
        n2925 = Build Array(FALSE, w4000, w3999, w3998, w3997, w3996, w3995, w3994, w3993, w3992, w3991, w3990, w3989, w3988, w3987, w3986, w3985, w3984, w3983, w3982, w3981, w3980, w3979, w3978, w3977, w3976, w3975, w3974, w3973, w3972, w3971) -> (w3970:bool[])
      }
      frame #5 {
        n2926 = local read "ch3-4 trns gv timer"() -> (w4451:bool)
        n2927 = local read "ch1-2 trns gv timer"() -> (w4450:bool)
        n2928 = local read "ch2-3 trns gv timer"() -> (w4456:bool)
        n2929 = local read "ch4 pc gv timer"() -> (w4492:bool)
        n2930 = local read "ch2 pc gv timer"() -> (w4493:bool)
        n2931 = local read "ch3 pc gv timer"() -> (w4487:bool)
        n2932 = local read "ch4 ch vbv timer"() -> (w4540:bool)
        n2933 = local read "ch1 pc gv timer"() -> (w4498:bool)
        n2934 = local read "ch2 ch vbv timer"() -> (w4541:bool)
        n2935 = local read "ch3 ch vbv timer"() -> (w4535:bool)
        n2936 = local read "ch4 bg bv timer"() -> (w4516:bool)
        n2937 = local read "ch1 ch vbv timer"() -> (w4546:bool)
        n2938 = local read "ch2 bg bv timer"() -> (w4517:bool)
        n2939 = local read "ch3 bg bv timer"() -> (w4511:bool)
        n2940 = local read "ch1 bg bv timer"() -> (w4522:bool)
        n2941 = local read "ch4 tp bv timer"() -> (w4564:bool)
        n2942 = local read "ch2 tp bv timer"() -> (w4565:bool)
        n2943 = local read "ch3 tp bv timer"() -> (w4559:bool)
        n2944 = local read "ch1 tp bv timer"() -> (w4570:bool)
        n2945 = local read "ch4 mp timer"() -> (w4588:bool)
        n2946 = local read "ch2 mp timer"() -> (w4589:bool)
        n2947 = local read "ch3 mp timer"() -> (w4583:bool)
        n2948 = local read "ch1 mp timer"() -> (w4594:bool)
        n2949 = feedback #85() -> (w4453:bool)  [unwired: 1 in]
        n2950 = feedback #86() -> (w4490:bool)  [unwired: 1 in]
        n2951 = feedback #87() -> (w4448:bool)  [unwired: 1 in]
        n2952 = feedback #88() -> (w4454:bool)  [unwired: 1 in]
        n2953 = feedback #89() -> (w4495:bool)  [unwired: 1 in]
        n2954 = feedback #90() -> (w4489:bool)  [unwired: 1 in]
        n2955 = feedback #91() -> (w4496:bool)  [unwired: 1 in]
        n2956 = feedback #92() -> (w4514:bool)  [unwired: 1 in]
        n2957 = feedback #93() -> (w4519:bool)  [unwired: 1 in]
        n2958 = feedback #94() -> (w4513:bool)  [unwired: 1 in]
        n2959 = feedback #95() -> (w4538:bool)  [unwired: 1 in]
        n2960 = feedback #96() -> (w4520:bool)  [unwired: 1 in]
        n2961 = feedback #97() -> (w4543:bool)  [unwired: 1 in]
        n2962 = feedback #98() -> (w4537:bool)  [unwired: 1 in]
        n2963 = feedback #99() -> (w4544:bool)  [unwired: 1 in]
        n2964 = feedback #100() -> (w4562:bool)  [unwired: 1 in]
        n2965 = feedback #101() -> (w4567:bool)  [unwired: 1 in]
        n2966 = feedback #102() -> (w4561:bool)  [unwired: 1 in]
        n2967 = feedback #103() -> (w4586:bool)  [unwired: 1 in]
        n2968 = feedback #104() -> (w4568:bool)  [unwired: 1 in]
        n2969 = feedback #105() -> (w4591:bool)  [unwired: 1 in]
        n2970 = feedback #106() -> (w4585:bool)  [unwired: 1 in]
        n2971 = feedback #107() -> (w4592:bool)  [unwired: 1 in]
        n2972 = case shown="True" w4451 {
          tunnel: [TRUE FALSE] -> w4452
          tunnel: w4453 -> [_ w4597]
          frame False {
          }
          frame True {
            n2973 = call "Elapsed Time57"("Auto Reset"=w4597) -> ("Elapsed Time (s)"=w4602:dbl)  [unwired: 11 in, 7 out]
            n2974 = Greater?(x=w4602, y=3.0) -> (0:w4599:bool)
            n2975 = In Range and Coerce(upper limit=3.0, x=w4602, lower limit=0.0 ("Elapsed Time (s)")) -> (In Range?=w4596:bool)  [unwired: 1 out]
            n2976 = Not(x=w4599) -> (.not. x?=w4598:bool)
            n2977 = property on="CH3-4 trnsgv timer tab" class="TabCtl (strict)"("Visible"=w4596) -> ()  [unwired: 2 in, 2 out]
            n2978 = local write "ch3-4 trns gv timer"(w4598) -> ()
          }
        }
        n2979 = feedback-in #85(w4452) -> ()
        n2980 = case shown="True" w4492 {
          tunnel: [TRUE FALSE] -> w4491
          tunnel: w4490 -> [_ w4727]
          frame False {
          }
          frame True {
            n2981 = call "Elapsed Time36"("Auto Reset"=w4727) -> ("Elapsed Time (s)"=w4732:dbl)  [unwired: 11 in, 7 out]
            n2982 = Greater?(x=w4732, y=3.0) -> (0:w4729:bool)
            n2983 = In Range and Coerce(upper limit=3.0, x=w4732, lower limit=0.0 ("Elapsed Time (s)")) -> (In Range?=w4726:bool)  [unwired: 1 out]
            n2984 = Not(x=w4729) -> (.not. x?=w4728:bool)
            n2985 = local write "ch4 pc gv timer"(w4728) -> ()
            n2986 = property on="pcgv4 timer tab" class="TabCtl (strict)"("Visible"=w4726) -> ()  [unwired: 2 in, 2 out]
          }
        }
        n2987 = feedback-in #86(w4491) -> ()
        n2988 = case shown="True" w4450 {
          tunnel: [TRUE FALSE] -> w4449
          tunnel: w4448 -> [_ w4617]
          frame False {
          }
          frame True {
            n2989 = call "Elapsed Time55"("Auto Reset"=w4617) -> ("Elapsed Time (s)"=w4622:dbl)  [unwired: 11 in, 7 out]
            n2990 = Greater?(x=w4622, y=3.0) -> (0:w4619:bool)
            n2991 = In Range and Coerce(upper limit=3.0, x=w4622, lower limit=0.0 ("Elapsed Time (s)")) -> (In Range?=w4616:bool)  [unwired: 1 out]
            n2992 = Not(x=w4619) -> (.not. x?=w4618:bool)
            n2993 = property on="CH1-2 trnsgv timer tab" class="TabCtl (strict)"("Visible"=w4616) -> ()  [unwired: 2 in, 2 out]
            n2994 = local write "ch1-2 trns gv timer"(w4618) -> ()
          }
        }
        n2995 = feedback-in #87(w4449) -> ()
        n2996 = case shown="True" w4456 {
          tunnel: [TRUE FALSE] -> w4455
          tunnel: w4454 -> [_ w4607]
          frame False {
          }
          frame True {
            n2997 = call "Elapsed Time56"("Auto Reset"=w4607) -> ("Elapsed Time (s)"=w4612:dbl)  [unwired: 11 in, 7 out]
            n2998 = Greater?(x=w4612, y=3.0) -> (0:w4609:bool)
            n2999 = In Range and Coerce(upper limit=3.0, x=w4612, lower limit=0.0 ("Elapsed Time (s)")) -> (In Range?=w4606:bool)  [unwired: 1 out]
            n3000 = Not(x=w4609) -> (.not. x?=w4608:bool)
            n3001 = property on="CH2-3 trnsgv timer tab" class="TabCtl (strict)"("Visible"=w4606) -> ()  [unwired: 2 in, 2 out]
            n3002 = local write "ch2-3 trns gv timer"(w4608) -> ()
          }
        }
        n3003 = feedback-in #88(w4455) -> ()
        n3004 = case shown="True" w4493 {
          tunnel: [TRUE FALSE] -> w4494
          tunnel: w4495 -> [_ w4747]
          frame False {
          }
          frame True {
            n3005 = call "Elapsed Time34"("Auto Reset"=w4747) -> ("Elapsed Time (s)"=w4752:dbl)  [unwired: 11 in, 7 out]
            n3006 = Greater?(x=w4752, y=3.0) -> (0:w4749:bool)
            n3007 = In Range and Coerce(upper limit=3.0, x=w4752, lower limit=0.0 ("Elapsed Time (s)")) -> (In Range?=w4746:bool)  [unwired: 1 out]
            n3008 = Not(x=w4749) -> (.not. x?=w4748:bool)
            n3009 = local write "ch2 pc gv timer"(w4748) -> ()
            n3010 = property on="pcgv2 timer tab" class="TabCtl (strict)"("Visible"=w4746) -> ()  [unwired: 2 in, 2 out]
          }
        }
        n3011 = feedback-in #89(w4494) -> ()
        n3012 = case shown="True" w4487 {
          tunnel: [TRUE FALSE] -> w4488
          tunnel: w4489 -> [_ w4737]
          frame False {
          }
          frame True {
            n3013 = call "Elapsed Time35"("Auto Reset"=w4737) -> ("Elapsed Time (s)"=w4742:dbl)  [unwired: 11 in, 7 out]
            n3014 = Greater?(x=w4742, y=3.0) -> (0:w4739:bool)
            n3015 = In Range and Coerce(upper limit=3.0, x=w4742, lower limit=0.0 ("Elapsed Time (s)")) -> (In Range?=w4736:bool)  [unwired: 1 out]
            n3016 = Not(x=w4739) -> (.not. x?=w4738:bool)
            n3017 = local write "ch3 pc gv timer"(w4738) -> ()
            n3018 = property on="pcgv3 timer tab" class="TabCtl (strict)"("Visible"=w4736) -> ()  [unwired: 2 in, 2 out]
          }
        }
        n3019 = feedback-in #90(w4488) -> ()
        n3020 = case shown="True" w4498 {
          tunnel: [TRUE FALSE] -> w4497
          tunnel: w4496 -> [_ w4757]
          frame False {
          }
          frame True {
            n3021 = call "Elapsed Time33"("Auto Reset"=w4757) -> ("Elapsed Time (s)"=w4762:dbl)  [unwired: 11 in, 7 out]
            n3022 = Greater?(x=w4762, y=3.0) -> (0:w4759:bool)
            n3023 = In Range and Coerce(upper limit=3.0, x=w4762, lower limit=0.0 ("Elapsed Time (s)")) -> (In Range?=w4756:bool)  [unwired: 1 out]
            n3024 = Not(x=w4759) -> (.not. x?=w4758:bool)
            n3025 = local write "ch1 pc gv timer"(w4758) -> ()
            n3026 = property on="pcgv1 timer tab" class="TabCtl (strict)"("Visible"=w4756) -> ()  [unwired: 2 in, 2 out]
          }
        }
        n3027 = feedback-in #91(w4497) -> ()
        n3028 = case shown="True" w4516 {
          tunnel: [TRUE FALSE] -> w4515
          tunnel: w4514 -> [_ w4807]
          frame False {
          }
          frame True {
            n3029 = call "Elapsed Time28"("Auto Reset"=w4807) -> ("Elapsed Time (s)"=w4812:dbl)  [unwired: 11 in, 7 out]
            n3030 = Greater?(x=w4812, y=3.0) -> (0:w4809:bool)
            n3031 = In Range and Coerce(upper limit=3.0, x=w4812, lower limit=0.0 ("Elapsed Time (s)")) -> (In Range?=w4806:bool)  [unwired: 1 out]
            n3032 = Not(x=w4809) -> (.not. x?=w4808:bool)
            n3033 = local write "ch4 bg bv timer"(w4808) -> ()
            n3034 = property on="bgbv4 timer tab" class="TabCtl (strict)"("Visible"=w4806) -> ()  [unwired: 2 in, 2 out]
          }
        }
        n3035 = feedback-in #92(w4515) -> ()
        n3036 = case shown="True" w4517 {
          tunnel: [TRUE FALSE] -> w4518
          tunnel: w4519 -> [_ w4827]
          frame False {
          }
          frame True {
            n3037 = call "Elapsed Time26"("Auto Reset"=w4827) -> ("Elapsed Time (s)"=w4832:dbl)  [unwired: 11 in, 7 out]
            n3038 = Greater?(x=w4832, y=3.0) -> (0:w4829:bool)
            n3039 = In Range and Coerce(upper limit=3.0, x=w4832, lower limit=0.0 ("Elapsed Time (s)")) -> (In Range?=w4826:bool)  [unwired: 1 out]
            n3040 = Not(x=w4829) -> (.not. x?=w4828:bool)
            n3041 = local write "ch2 bg bv timer"(w4828) -> ()
            n3042 = property on="bgbv2 timer tab" class="TabCtl (strict)"("Visible"=w4826) -> ()  [unwired: 2 in, 2 out]
          }
        }
        n3043 = feedback-in #93(w4518) -> ()
        n3044 = case shown="True" w4511 {
          tunnel: [TRUE FALSE] -> w4512
          tunnel: w4513 -> [_ w4817]
          frame False {
          }
          frame True {
            n3045 = call "Elapsed Time27"("Auto Reset"=w4817) -> ("Elapsed Time (s)"=w4822:dbl)  [unwired: 11 in, 7 out]
            n3046 = Greater?(x=w4822, y=3.0) -> (0:w4819:bool)
            n3047 = In Range and Coerce(upper limit=3.0, x=w4822, lower limit=0.0 ("Elapsed Time (s)")) -> (In Range?=w4816:bool)  [unwired: 1 out]
            n3048 = Not(x=w4819) -> (.not. x?=w4818:bool)
            n3049 = local write "ch3 bg bv timer"(w4818) -> ()
            n3050 = property on="bgbv3 timer tab" class="TabCtl (strict)"("Visible"=w4816) -> ()  [unwired: 2 in, 2 out]
          }
        }
        n3051 = feedback-in #94(w4512) -> ()
        n3052 = case shown="True" w4540 {
          tunnel: [TRUE FALSE] -> w4539
          tunnel: w4538 -> [_ w4883]
          frame False {
          }
          frame True {
            n3053 = call "Elapsed Time20"("Auto Reset"=w4883) -> ("Elapsed Time (s)"=w4888:dbl)  [unwired: 11 in, 7 out]
            n3054 = Greater?(x=w4888, y=3.0) -> (0:w4885:bool)
            n3055 = In Range and Coerce(upper limit=3.0, x=w4888, lower limit=0.0 ("Elapsed Time (s)")) -> (In Range?=w4882:bool)  [unwired: 1 out]
            n3056 = Not(x=w4885) -> (.not. x?=w4884:bool)
            n3057 = local write "ch4 ch vbv timer"(w4884) -> ()
            n3058 = property on="chvbv4 timer tab" class="TabCtl (strict)"("Visible"=w4882) -> ()  [unwired: 2 in, 2 out]
          }
        }
        n3059 = feedback-in #95(w4539) -> ()
        n3060 = case shown="True" w4522 {
          tunnel: [TRUE FALSE] -> w4521
          tunnel: w4520 -> [_ w4837]
          frame False {
          }
          frame True {
            n3061 = call "Elapsed Time25"("Auto Reset"=w4837) -> ("Elapsed Time (s)"=w4842:dbl)  [unwired: 11 in, 7 out]
            n3062 = Greater?(x=w4842, y=3.0) -> (0:w4839:bool)
            n3063 = In Range and Coerce(upper limit=3.0, x=w4842, lower limit=0.0 ("Elapsed Time (s)")) -> (In Range?=w4836:bool)  [unwired: 1 out]
            n3064 = Not(x=w4839) -> (.not. x?=w4838:bool)
            n3065 = local write "ch1 bg bv timer"(w4838) -> ()
            n3066 = property on="bgbv1 timer tab" class="TabCtl (strict)"("Visible"=w4836) -> ()  [unwired: 2 in, 2 out]
          }
        }
        n3067 = feedback-in #96(w4521) -> ()
        n3068 = case shown="True" w4541 {
          tunnel: [TRUE FALSE] -> w4542
          tunnel: w4543 -> [_ w4903]
          frame False {
          }
          frame True {
            n3069 = call "Elapsed Time18"("Auto Reset"=w4903) -> ("Elapsed Time (s)"=w4908:dbl)  [unwired: 11 in, 7 out]
            n3070 = Greater?(x=w4908, y=3.0) -> (0:w4905:bool)
            n3071 = In Range and Coerce(upper limit=3.0, x=w4908, lower limit=0.0 ("Elapsed Time (s)")) -> (In Range?=w4902:bool)  [unwired: 1 out]
            n3072 = Not(x=w4905) -> (.not. x?=w4904:bool)
            n3073 = local write "ch2 ch vbv timer"(w4904) -> ()
            n3074 = property on="chvbv2 timer tab" class="TabCtl (strict)"("Visible"=w4902) -> ()  [unwired: 2 in, 2 out]
          }
        }
        n3075 = feedback-in #97(w4542) -> ()
        n3076 = case shown="True" w4535 {
          tunnel: [TRUE FALSE] -> w4536
          tunnel: w4537 -> [_ w4893]
          frame False {
          }
          frame True {
            n3077 = call "Elapsed Time19"("Auto Reset"=w4893) -> ("Elapsed Time (s)"=w4898:dbl)  [unwired: 11 in, 7 out]
            n3078 = Greater?(x=w4898, y=3.0) -> (0:w4895:bool)